vi "FlexMag - 23-03-2023.vi"() -> ()   [LabVIEW 2018] (continued)
                                n20029 = Greater?(x=w24311, y=0.0) -> (0:w24310:bool)
                                n20030 = case shown="True" w24310 {
                                frame False {
                                }
                                frame True {
                                n20031 = flat-sequence {
                                frame #0 {
                                n20032 = local read "R dc step length 5"() -> (w24318:dbl)
                                n20033 = local read "R dc step power 5"() -> (w24313:dbl)
                                n20034 = local read "R web speed"() -> (w24317:dbl)
                                n20035 = Divide(x=w24318, y=w24317) -> (x/y=w24316:dbl)
                                n20036 = Wait (ms)(milliseconds to wait=u32 100) -> ()  [unwired: 1 out]
                                n20037 = local write "Set DC Power ch2"(w24313) -> ()
                                n20038 = Multiply(x=w24316, y=60) -> (x*y=w24314:dbl)
                                n20039 = local write "time counting"(w24314) -> ()
                                }
                                frame #1 {
                                n20040 = local write "Dc_auto_set"(TRUE ("Dc_auto_set")) -> ()
                                }
                                frame #2 {
                                n20041 = while {
                                stop <- w24321 stop-if-true
                                n20042 = local read "time counting"() -> (w24327:dbl)
                                n20043 = local read "coating start"() -> (w24325:bool)
                                n20044 = Wait Until Next ms Multiple(millisecond multiple=u32 1000) -> ()  [unwired: 1 out]
                                n20045 = local read "abort ch2"() -> (w24323:bool)
                                n20046 = Decrement(x=w24327) -> (x-1=w24326:dbl)
                                n20047 = local write "time counting"(w24326) -> ()
                                n20048 = Not(x=w24325) -> (.not. x?=w24324:bool)
                                n20049 = Less Or Equal To 0?(x=w24326) -> (x <= 0?=w24322:bool)
                                n20050 = Compound Arithmetic op=OR(w24322, w24324, w24323) -> (w24321:bool)
                                }
                                }
                                }
                                }
                                }
                                }
                                }
                                }
                                frame True {
                                }
                                }
                                }
                                frame #5 {
                                n20051 = local read "abort ch2"() -> (w24328:bool)
                                n20052 = case shown="False" w24328 {
                                frame False {
                                n20053 = local read "coating start"() -> (w24329:bool)
                                n20054 = case shown="True" w24329 {
                                frame False {
                                }
                                frame True {
                                n20055 = local read "R dc step length 6"() -> (w24332:dbl)
                                n20056 = Greater?(x=w24332, y=0.0) -> (0:w24331:bool)
                                n20057 = case shown="True" w24331 {
                                frame False {
                                }
                                frame True {
                                n20058 = flat-sequence {
                                frame #0 {
                                n20059 = local read "R dc step length 6"() -> (w24339:dbl)
                                n20060 = local read "R dc step power 6"() -> (w24334:dbl)
                                n20061 = local read "R web speed"() -> (w24338:dbl)
                                n20062 = Wait (ms)(milliseconds to wait=u32 100) -> ()  [unwired: 1 out]
                                n20063 = Divide(x=w24339, y=w24338) -> (x/y=w24337:dbl)
                                n20064 = local write "Set DC Power ch2"(w24334) -> ()
                                n20065 = Multiply(x=w24337, y=60) -> (x*y=w24335:dbl)
                                n20066 = local write "time counting"(w24335) -> ()
                                }
                                frame #1 {
                                n20067 = local write "Dc_auto_set"(TRUE ("Dc_auto_set")) -> ()
                                }
                                frame #2 {
                                n20068 = while {
                                stop <- w24342 stop-if-true
                                n20069 = local read "time counting"() -> (w24348:dbl)
                                n20070 = local read "coating start"() -> (w24346:bool)
                                n20071 = local read "abort ch2"() -> (w24344:bool)
                                n20072 = Wait Until Next ms Multiple(millisecond multiple=u32 1000) -> ()  [unwired: 1 out]
                                n20073 = Decrement(x=w24348) -> (x-1=w24347:dbl)
                                n20074 = local write "time counting"(w24347) -> ()
                                n20075 = Not(x=w24346) -> (.not. x?=w24345:bool)
                                n20076 = Less Or Equal To 0?(x=w24347) -> (x <= 0?=w24343:bool)
                                n20077 = Compound Arithmetic op=OR(w24343, w24345, w24344) -> (w24342:bool)
                                }
                                }
                                }
                                }
                                }
                                }
                                }
                                }
                                frame True {
                                }
                                }
                                }
                                frame #6 {
                                n20078 = local read "abort ch2"() -> (w24349:bool)
                                n20079 = case shown="False" w24349 {
                                frame False {
                                n20080 = local read "coating start"() -> (w24350:bool)
                                n20081 = case shown="True" w24350 {
                                frame False {
                                }
                                frame True {
                                n20082 = local read "R dc step length 7"() -> (w24353:dbl)
                                n20083 = Greater?(x=w24353, y=0.0) -> (0:w24352:bool)
                                n20084 = case shown="True" w24352 {
                                frame False {
                                }
                                frame True {
                                n20085 = flat-sequence {
                                frame #0 {
                                n20086 = local read "R dc step length 7"() -> (w24360:dbl)
                                n20087 = local read "R dc step power 7"() -> (w24355:dbl)
                                n20088 = local read "R web speed"() -> (w24359:dbl)
                                n20089 = Divide(x=w24360, y=w24359) -> (x/y=w24358:dbl)
                                n20090 = Wait (ms)(milliseconds to wait=u32 100) -> ()  [unwired: 1 out]
                                n20091 = local write "Set DC Power ch2"(w24355) -> ()
                                n20092 = Multiply(x=w24358, y=60) -> (x*y=w24356:dbl)
                                n20093 = local write "time counting"(w24356) -> ()
                                }
                                frame #1 {
                                n20094 = local write "Dc_auto_set"(TRUE ("Dc_auto_set")) -> ()
                                }
                                frame #2 {
                                n20095 = while {
                                stop <- w24363 stop-if-true
                                n20096 = local read "time counting"() -> (w24369:dbl)
                                n20097 = local read "coating start"() -> (w24367:bool)
                                n20098 = local read "abort ch2"() -> (w24365:bool)
                                n20099 = Wait Until Next ms Multiple(millisecond multiple=u32 1000) -> ()  [unwired: 1 out]
                                n20100 = Decrement(x=w24369) -> (x-1=w24368:dbl)
                                n20101 = local write "time counting"(w24368) -> ()
                                n20102 = Not(x=w24367) -> (.not. x?=w24366:bool)
                                n20103 = Less Or Equal To 0?(x=w24368) -> (x <= 0?=w24364:bool)
                                n20104 = Compound Arithmetic op=OR(w24364, w24366, w24365) -> (w24363:bool)
                                }
                                }
                                }
                                }
                                }
                                }
                                }
                                }
                                frame True {
                                }
                                }
                                }
                                frame #7 {
                                n20105 = local read "abort ch2"() -> (w24370:bool)
                                n20106 = case shown="False" w24370 {
                                frame False {
                                n20107 = local read "coating start"() -> (w24371:bool)
                                n20108 = case shown="True" w24371 {
                                frame False {
                                }
                                frame True {
                                n20109 = local read "R dc step length 8"() -> (w24374:dbl)
                                n20110 = Greater?(x=w24374, y=0.0) -> (0:w24373:bool)
                                n20111 = case shown="True" w24373 {
                                frame False {
                                }
                                frame True {
                                n20112 = flat-sequence {
                                frame #0 {
                                n20113 = local read "R dc step length 8"() -> (w24381:dbl)
                                n20114 = local read "R dc step power 8"() -> (w24376:dbl)
                                n20115 = local read "R web speed"() -> (w24380:dbl)
                                n20116 = Wait (ms)(milliseconds to wait=u32 100) -> ()  [unwired: 1 out]
                                n20117 = Divide(x=w24381, y=w24380) -> (x/y=w24379:dbl)
                                n20118 = local write "Set DC Power ch2"(w24376) -> ()
                                n20119 = Multiply(x=w24379, y=60) -> (x*y=w24377:dbl)
                                n20120 = local write "time counting"(w24377) -> ()
                                }
                                frame #1 {
                                n20121 = local write "Dc_auto_set"(TRUE ("Dc_auto_set")) -> ()
                                }
                                frame #2 {
                                n20122 = while {
                                stop <- w24384 stop-if-true
                                n20123 = local read "time counting"() -> (w24390:dbl)
                                n20124 = local read "coating start"() -> (w24388:bool)
                                n20125 = Wait Until Next ms Multiple(millisecond multiple=u32 1000) -> ()  [unwired: 1 out]
                                n20126 = local read "abort ch2"() -> (w24386:bool)
                                n20127 = Decrement(x=w24390) -> (x-1=w24389:dbl)
                                n20128 = local write "time counting"(w24389) -> ()
                                n20129 = Not(x=w24388) -> (.not. x?=w24387:bool)
                                n20130 = Less Or Equal To 0?(x=w24389) -> (x <= 0?=w24385:bool)
                                n20131 = Compound Arithmetic op=OR(w24385, w24387, w24386) -> (w24384:bool)
                                }
                                }
                                }
                                }
                                }
                                }
                                }
                                }
                                frame True {
                                }
                                }
                                }
                                frame #8 {
                                n20132 = local read "abort ch2"() -> (w24391:bool)
                                n20133 = case shown="False" w24391 {
                                frame False {
                                n20134 = local read "coating start"() -> (w24392:bool)
                                n20135 = case shown="True" w24392 {
                                frame False {
                                }
                                frame True {
                                n20136 = local read "R dc step length 9"() -> (w24395:dbl)
                                n20137 = Greater?(x=w24395, y=0.0) -> (0:w24394:bool)
                                n20138 = case shown="True" w24394 {
                                frame False {
                                }
                                frame True {
                                n20139 = flat-sequence {
                                frame #0 {
                                n20140 = local read "R dc step length 9"() -> (w24402:dbl)
                                n20141 = local read "R dc step power 9"() -> (w24397:dbl)
                                n20142 = local read "R web speed"() -> (w24401:dbl)
                                n20143 = Wait (ms)(milliseconds to wait=u32 100) -> ()  [unwired: 1 out]
                                n20144 = Divide(x=w24402, y=w24401) -> (x/y=w24400:dbl)
                                n20145 = local write "Set DC Power ch2"(w24397) -> ()
                                n20146 = Multiply(x=w24400, y=60) -> (x*y=w24398:dbl)
                                n20147 = local write "time counting"(w24398) -> ()
                                }
                                frame #1 {
                                n20148 = local write "Dc_auto_set"(TRUE ("Dc_auto_set")) -> ()
                                }
                                frame #2 {
                                n20149 = while {
                                stop <- w24405 stop-if-true
                                n20150 = local read "time counting"() -> (w24411:dbl)
                                n20151 = local read "coating start"() -> (w24409:bool)
                                n20152 = local read "abort ch2"() -> (w24407:bool)
                                n20153 = Wait Until Next ms Multiple(millisecond multiple=u32 1000) -> ()  [unwired: 1 out]
                                n20154 = Decrement(x=w24411) -> (x-1=w24410:dbl)
                                n20155 = local write "time counting"(w24410) -> ()
                                n20156 = Not(x=w24409) -> (.not. x?=w24408:bool)
                                n20157 = Less Or Equal To 0?(x=w24410) -> (x <= 0?=w24406:bool)
                                n20158 = Compound Arithmetic op=OR(w24406, w24408, w24407) -> (w24405:bool)
                                }
                                }
                                }
                                }
                                }
                                }
                                }
                                }
                                frame True {
                                }
                                }
                                }
                                frame #9 {
                                n20159 = local read "abort ch2"() -> (w24412:bool)
                                n20160 = case shown="False" w24412 {
                                frame False {
                                n20161 = local read "coating start"() -> (w24413:bool)
                                n20162 = case shown="True" w24413 {
                                frame False {
                                }
                                frame True {
                                n20163 = local read "R dc step length 10"() -> (w24416:dbl)
                                n20164 = Greater?(x=w24416, y=0.0) -> (0:w24415:bool)
                                n20165 = case shown="True" w24415 {
                                frame False {
                                }
                                frame True {
                                n20166 = flat-sequence {
                                frame #0 {
                                n20167 = local read "R dc step length 10"() -> (w24423:dbl)
                                n20168 = local read "R dc step power 10"() -> (w24418:dbl)
                                n20169 = local read "R web speed"() -> (w24422:dbl)
                                n20170 = Divide(x=w24423, y=w24422) -> (x/y=w24421:dbl)
                                n20171 = local write "Set DC Power ch2"(w24418) -> ()
                                n20172 = Wait (ms)(milliseconds to wait=u32 100) -> ()  [unwired: 1 out]
                                n20173 = Multiply(x=w24421, y=60) -> (x*y=w24419:dbl)
                                n20174 = local write "time counting"(w24419) -> ()
                                }
                                frame #1 {
                                n20175 = local write "Dc_auto_set"(TRUE ("Dc_auto_set")) -> ()
                                }
                                frame #2 {
                                n20176 = while {
                                stop <- w24426 stop-if-true
                                n20177 = local read "time counting"() -> (w24432:dbl)
                                n20178 = local read "coating start"() -> (w24430:bool)
                                n20179 = local read "abort ch2"() -> (w24428:bool)
                                n20180 = Wait Until Next ms Multiple(millisecond multiple=u32 1000) -> ()  [unwired: 1 out]
                                n20181 = Decrement(x=w24432) -> (x-1=w24431:dbl)
                                n20182 = local write "time counting"(w24431) -> ()
                                n20183 = Not(x=w24430) -> (.not. x?=w24429:bool)
                                n20184 = Less Or Equal To 0?(x=w24431) -> (x <= 0?=w24427:bool)
                                n20185 = Compound Arithmetic op=OR(w24427, w24429, w24428) -> (w24426:bool)
                                }
                                }
                                }
                                }
                                }
                                }
                                }
                                }
                                frame True {
                                }
                                }
                                }
                                frame #10 {
                                n20186 = local read "abort ch2"() -> (w24433:bool)
                                n20187 = case shown="False" w24433 {
                                frame False {
                                n20188 = local read "coating start"() -> (w24434:bool)
                                n20189 = case shown="True" w24434 {
                                frame False {
                                }
                                frame True {
                                n20190 = Wait (ms)(milliseconds to wait=u32 100) -> ()  [unwired: 1 out]
                                "coating ch2 led 12" <- TRUE ("coating ch2 led 1")
                                }
                                }
                                }
                                frame True {
                                }
                                }
                                }
                                }
                                }
                                frame Enabled {
                                n20191 = stacked-sequence {
                                frame #0 {
                                n20192 = local read "abort ch2"() -> (w24437:bool)
                                n20193 = case shown="False" w24437 {
                                frame False {
                                n20194 = local read "coating start"() -> (w24438:bool)
                                n20195 = case shown="True" w24438 {
                                frame False {
                                }
                                frame True {
                                n20196 = local read "dep. for?"() -> (w24439:bool)
                                n20197 = case shown="True" w24439 {
                                frame False {
                                n20198 = flat-sequence {
                                frame #0 {
                                n20199 = local read "R DC number steps"() -> (w24442:dbl)
                                n20200 = case shown="10" w24442 {
                                tunnel: [0.0 ("step up") 1.0 ("step up") 2.0 ("step up") 3.0 ("step up") 4.0 ("step up") 5.0 ("step up") 6.0 ("step up") 7.0 ("step up") 8.0 ("step up") 9.0 ("step up") 10.0 ("step up") 11.0 ("step up") 12.0 ("step up") 13.0 ("step up") 14.0 ("step up") 15.0 ("step up") 16.0 ("step up") 17.0 ("step up") 18.0 ("step up") 19.0 ("step up") 20.0 ("step up")] -> w24441
                                tunnel: [200.0 ("R dc step power 1") w24447 w24449 w24451 w24453 w24455 w24457 w24459 w24461 w24463 w24465 w24467 w24469 w24471 w24473 w24475 w24477 w24479 w24481 w24483 w24485] -> w24440
                                frame 0, Default {
                                }
                                frame 1 {
                                n20201 = local read "R dc step power 1"() -> (w24447:dbl)
                                }
                                frame 2 {
                                n20202 = local read "R dc step power 2"() -> (w24449:dbl)
                                }
                                frame 3 {
                                n20203 = local read "R dc step power 3"() -> (w24451:dbl)
                                }
                                frame 4 {
                                n20204 = local read "R dc step power 4"() -> (w24453:dbl)
                                }
                                frame 5 {
                                n20205 = local read "R dc step power 5"() -> (w24455:dbl)
                                }
                                frame 6 {
                                n20206 = local read "R dc step power 6"() -> (w24457:dbl)
                                }
                                frame 7 {
                                n20207 = local read "R dc step power 7"() -> (w24459:dbl)
                                }
                                frame 8 {
                                n20208 = local read "R dc step power 8"() -> (w24461:dbl)
                                }
                                frame 9 {
                                n20209 = local read "R dc step power 9"() -> (w24463:dbl)
                                }
                                frame 10 {
                                n20210 = local read "R dc step power 10"() -> (w24465:dbl)
                                }
                                frame 11 {
                                n20211 = local read "R dc step power 11"() -> (w24467:dbl)
                                }
                                frame 12 {
                                n20212 = local read "R dc step power 12"() -> (w24469:dbl)
                                }
                                frame 13 {
                                n20213 = local read "R dc step power 13"() -> (w24471:dbl)
                                }
                                frame 14 {
                                n20214 = local read "R dc step power 14"() -> (w24473:dbl)
                                }
                                frame 15 {
                                n20215 = local read "R dc step power 15"() -> (w24475:dbl)
                                }
                                frame 16 {
                                n20216 = local read "R dc step power 16"() -> (w24477:dbl)
                                }
                                frame 17 {
                                n20217 = local read "R dc step power 17"() -> (w24479:dbl)
                                }
                                frame 18 {
                                n20218 = local read "R dc step power 18"() -> (w24481:dbl)
                                }
                                frame 19 {
                                n20219 = local read "R dc step power 19"() -> (w24483:dbl)
                                }
                                frame 20 {
                                n20220 = local read "R dc step power 20"() -> (w24485:dbl)
                                }
                                }
                                n20221 = Wait (ms)(milliseconds to wait=u32 100) -> ()  [unwired: 1 out]
                                n20222 = local write "current step"(w24441) -> ()
                                n20223 = local write "Set DC Power auto"(w24440) -> ()
                                }
                                frame #1 {
                                n20224 = local write "Dc_auto_set"(TRUE ("Dc_auto_set")) -> ()
                                }
                                frame #2 {
                                n20225 = Wait (ms)(milliseconds to wait=u32 1000) -> ()  [unwired: 1 out]
                                }
                                }
                                }
                                frame True {
                                n20226 = flat-sequence {
                                frame #0 {
                                n20227 = local read "R dc step power 1"() -> (w24490:dbl)
                                n20228 = Wait (ms)(milliseconds to wait=u32 100) -> ()  [unwired: 1 out]
                                n20229 = local write "Set DC Power auto"(w24490) -> ()
                                n20230 = local write "current step"(1.0 ("step up")) -> ()
                                }
                                frame #1 {
                                n20231 = local write "Dc_auto_set"(TRUE ("Dc_auto_set")) -> ()
                                }
                                frame #2 {
                                n20232 = Wait (ms)(milliseconds to wait=u32 1000) -> ()  [unwired: 1 out]
                                }
                                }
                                }
                                }
                                }
                                }
                                }
                                frame True {
                                }
                                }
                                }
                                frame #1 {
                                n20233 = local read "abort ch2"() -> (w24493:bool)
                                n20234 = case shown="False" w24493 {
                                frame False {
                                n20235 = local read "coating start"() -> (w24494:bool)
                                n20236 = case shown="True" w24494 {
                                frame False {
                                }
                                frame True {
                                n20237 = while {
                                i -> [w24495]
                                stop <- w24507 stop-if-true
                                n20238 = local read "step count"() -> (w24510:dbl)
                                n20239 = local read "R DC number steps"() -> (w24508:dbl)
                                n20240 = local read "roll error (min)"() -> (w24498:i32)
                                n20241 = Wait Until Next ms Multiple(millisecond multiple=u32 300) -> ()  [unwired: 1 out]
                                n20242 = feedback #340() -> (w24511:dbl)  [unwired: 1 in]
                                n20243 = feedback-in #340(w24510) -> ()
                                n20244 = Multiply(x=200, y=w24498) -> (x*y=w24499:i32)
                                n20245 = Less?(x=w24510, y=w24511) -> (x < y?=w24509:bool)
                                n20246 = case shown="True" w24509 {
                                tunnel: w24508 -> [_ w24518]
                                tunnel: [FALSE w24515] -> w24501
                                frame False {
                                }
                                frame True {
                                n20247 = local read "current step"() -> (w24517:dbl)
                                n20248 = Greater Or Equal?(x=w24518, y=w24517) -> (x >= y?=w24516:bool)
                                n20249 = Not(x=w24516) -> (.not. x?=w24515:bool)
                                n20250 = case shown="True" w24516 {
                                tunnel: w24517 -> [_ w24519]
                                frame False {
                                }
                                frame True {
                                n20251 = case shown="4" w24519 {
                                frame 0, Default {
                                }
                                frame 1 {
                                n20252 = stacked-sequence {
                                frame #0 {
                                n20253 = local read "R dc step power 1"() -> (w24521:dbl)
                                n20254 = local write "Set DC Power auto"(w24521) -> ()
                                n20255 = Wait (ms)(milliseconds to wait=u32 100) -> ()  [unwired: 1 out]
                                }
                                frame #1 {
                                n20256 = local write "Dc_auto_set"(TRUE ("Dc_auto_set")) -> ()
                                }
                                }
                                }
                                frame 2 {
                                n20257 = stacked-sequence {
                                frame #0 {
                                n20258 = local read "R dc step power 2"() -> (w24524:dbl)
                                n20259 = local write "Set DC Power auto"(w24524) -> ()
                                n20260 = Wait (ms)(milliseconds to wait=u32 100) -> ()  [unwired: 1 out]
                                }
                                frame #1 {
                                n20261 = local write "Dc_auto_set"(TRUE ("Dc_auto_set")) -> ()
                                }
                                }
                                }
                                frame 3 {
                                n20262 = stacked-sequence {
                                frame #0 {
                                n20263 = local read "R dc step power 3"() -> (w24527:dbl)
                                n20264 = local write "Set DC Power auto"(w24527) -> ()
                                n20265 = Wait (ms)(milliseconds to wait=u32 100) -> ()  [unwired: 1 out]
                                }
                                frame #1 {
                                n20266 = local write "Dc_auto_set"(TRUE ("Dc_auto_set")) -> ()
                                }
                                }
                                }
                                frame 4 {
                                n20267 = stacked-sequence {
                                frame #0 {
                                n20268 = local read "R dc step power 4"() -> (w24530:dbl)
                                n20269 = local write "Set DC Power auto"(w24530) -> ()
                                n20270 = Wait (ms)(milliseconds to wait=u32 100) -> ()  [unwired: 1 out]
                                }
                                frame #1 {
                                n20271 = local write "Dc_auto_set"(TRUE ("Dc_auto_set")) -> ()
                                }
                                }
                                }
                                frame 5 {
                                n20272 = stacked-sequence {
                                frame #0 {
                                n20273 = local read "R dc step power 5"() -> (w24533:dbl)
                                n20274 = local write "Set DC Power auto"(w24533) -> ()
                                n20275 = Wait (ms)(milliseconds to wait=u32 100) -> ()  [unwired: 1 out]
                                }
                                frame #1 {
                                n20276 = local write "Dc_auto_set"(TRUE ("Dc_auto_set")) -> ()
                                }
                                }
                                }
                                frame 6 {
                                n20277 = stacked-sequence {
                                frame #0 {
                                n20278 = local read "R dc step power 6"() -> (w24536:dbl)
                                n20279 = local write "Set DC Power auto"(w24536) -> ()
                                n20280 = Wait (ms)(milliseconds to wait=u32 100) -> ()  [unwired: 1 out]
                                }
                                frame #1 {
                                n20281 = local write "Dc_auto_set"(TRUE ("Dc_auto_set")) -> ()
                                }
                                }
                                }
                                frame 7 {
                                n20282 = stacked-sequence {
                                frame #0 {
                                n20283 = local read "R dc step power 7"() -> (w24539:dbl)
                                n20284 = local write "Set DC Power auto"(w24539) -> ()
                                n20285 = Wait (ms)(milliseconds to wait=u32 100) -> ()  [unwired: 1 out]
                                }
                                frame #1 {
                                n20286 = local write "Dc_auto_set"(TRUE ("Dc_auto_set")) -> ()
                                }
                                }
                                }
                                frame 8 {
                                n20287 = stacked-sequence {
                                frame #0 {
                                n20288 = local read "R dc step power 8"() -> (w24542:dbl)
                                n20289 = local write "Set DC Power auto"(w24542) -> ()
                                n20290 = Wait (ms)(milliseconds to wait=u32 100) -> ()  [unwired: 1 out]
                                }
                                frame #1 {
                                n20291 = local write "Dc_auto_set"(TRUE ("Dc_auto_set")) -> ()
                                }
                                }
                                }
                                frame 9 {
                                n20292 = stacked-sequence {
                                frame #0 {
                                n20293 = local read "R dc step power 9"() -> (w24545:dbl)
                                n20294 = local write "Set DC Power auto"(w24545) -> ()
                                n20295 = Wait (ms)(milliseconds to wait=u32 100) -> ()  [unwired: 1 out]
                                }
                                frame #1 {
                                n20296 = local write "Dc_auto_set"(TRUE ("Dc_auto_set")) -> ()
                                }
                                }
                                }
                                frame 10 {
                                n20297 = stacked-sequence {
                                frame #0 {
                                n20298 = local read "R dc step power 10"() -> (w24548:dbl)
                                n20299 = local write "Set DC Power auto"(w24548) -> ()
                                n20300 = Wait (ms)(milliseconds to wait=u32 100) -> ()  [unwired: 1 out]
                                }
                                frame #1 {
                                n20301 = local write "Dc_auto_set"(TRUE ("Dc_auto_set")) -> ()
                                }
                                }
                                }
                                frame 11 {
                                n20302 = stacked-sequence {
                                frame #0 {
                                n20303 = local read "R dc step power 11"() -> (w24551:dbl)
                                n20304 = local write "Set DC Power auto"(w24551) -> ()
                                n20305 = Wait (ms)(milliseconds to wait=u32 100) -> ()  [unwired: 1 out]
                                }
                                frame #1 {
                                n20306 = local write "Dc_auto_set"(TRUE ("Dc_auto_set")) -> ()
                                }
                                }
                                }
                                frame 12 {
                                n20307 = stacked-sequence {
                                frame #0 {
                                n20308 = local read "R dc step power 12"() -> (w24554:dbl)
                                n20309 = local write "Set DC Power auto"(w24554) -> ()
                                n20310 = Wait (ms)(milliseconds to wait=u32 100) -> ()  [unwired: 1 out]
                                }
                                frame #1 {
                                n20311 = local write "Dc_auto_set"(TRUE ("Dc_auto_set")) -> ()
                                }
                                }
                                }
                                frame 13 {
                                n20312 = stacked-sequence {
                                frame #0 {
                                n20313 = local read "R dc step power 13"() -> (w24557:dbl)
                                n20314 = local write "Set DC Power auto"(w24557) -> ()
                                n20315 = Wait (ms)(milliseconds to wait=u32 100) -> ()  [unwired: 1 out]
                                }
                                frame #1 {
                                n20316 = local write "Dc_auto_set"(TRUE ("Dc_auto_set")) -> ()
                                }
                                }
                                }
                                frame 14 {
                                n20317 = stacked-sequence {
                                frame #0 {
                                n20318 = local read "R dc step power 14"() -> (w24560:dbl)
                                n20319 = local write "Set DC Power auto"(w24560) -> ()
                                n20320 = Wait (ms)(milliseconds to wait=u32 100) -> ()  [unwired: 1 out]
                                }
                                frame #1 {
                                n20321 = local write "Dc_auto_set"(TRUE ("Dc_auto_set")) -> ()
                                }
                                }
                                }
                                frame 15 {
                                n20322 = stacked-sequence {
                                frame #0 {
                                n20323 = local read "R dc step power 15"() -> (w24563:dbl)
                                n20324 = local write "Set DC Power auto"(w24563) -> ()
                                n20325 = Wait (ms)(milliseconds to wait=u32 100) -> ()  [unwired: 1 out]
                                }
                                frame #1 {
                                n20326 = local write "Dc_auto_set"(TRUE ("Dc_auto_set")) -> ()
                                }
                                }
                                }
                                frame 16 {
                                n20327 = stacked-sequence {
                                frame #0 {
                                n20328 = local read "R dc step power 16"() -> (w24566:dbl)
                                n20329 = local write "Set DC Power auto"(w24566) -> ()
                                n20330 = Wait (ms)(milliseconds to wait=u32 100) -> ()  [unwired: 1 out]
                                }
                                frame #1 {
                                n20331 = local write "Dc_auto_set"(TRUE ("Dc_auto_set")) -> ()
                                }
                                }
                                }
                                frame 17 {
                                n20332 = stacked-sequence {
                                frame #0 {
                                n20333 = local read "R dc step power 17"() -> (w24569:dbl)
                                n20334 = local write "Set DC Power auto"(w24569) -> ()
                                n20335 = Wait (ms)(milliseconds to wait=u32 100) -> ()  [unwired: 1 out]
                                }
                                frame #1 {
                                n20336 = local write "Dc_auto_set"(TRUE ("Dc_auto_set")) -> ()
                                }
                                }
                                }
                                frame 18 {
                                n20337 = stacked-sequence {
                                frame #0 {
                                n20338 = local read "R dc step power 18"() -> (w24572:dbl)
                                n20339 = local write "Set DC Power auto"(w24572) -> ()
                                n20340 = Wait (ms)(milliseconds to wait=u32 100) -> ()  [unwired: 1 out]
                                }
                                frame #1 {
                                n20341 = local write "Dc_auto_set"(TRUE ("Dc_auto_set")) -> ()
                                }
                                }
                                }
                                frame 19 {
                                n20342 = stacked-sequence {
                                frame #0 {
                                n20343 = local read "R dc step power 19"() -> (w24575:dbl)
                                n20344 = local write "Set DC Power auto"(w24575) -> ()
                                n20345 = Wait (ms)(milliseconds to wait=u32 100) -> ()  [unwired: 1 out]
                                }
                                frame #1 {
                                n20346 = local write "Dc_auto_set"(TRUE ("Dc_auto_set")) -> ()
                                }
                                }
                                }
                                frame 20 {
                                n20347 = stacked-sequence {
                                frame #0 {
                                n20348 = local read "R dc step power 20"() -> (w24578:dbl)
                                n20349 = local write "Set DC Power auto"(w24578) -> ()
                                n20350 = Wait (ms)(milliseconds to wait=u32 100) -> ()  [unwired: 1 out]
                                }
                                frame #1 {
                                n20351 = local write "Dc_auto_set"(TRUE ("Dc_auto_set")) -> ()
                                }
                                }
                                }
                                }
                                }
                                }
                                }
                                }
                                n20352 = Greater?(x=w24495, y=w24499) -> (0:w24497:bool)
                                n20353 = case shown="True" w24497 {
                                frame False {
                                }
                                frame True {
                                n20354 = local write "Warning Message"("Automatic Coating Process is canceled !\nCH2  rolling problem..." ("Warning Message")) -> ()
                                n20355 = local write "coating error"(TRUE ("coating error")) -> ()
                                }
                                }
                                n20356 = local read "CH2_Motor DO"() -> (w24503:bool)
                                n20357 = local read "coating start"() -> (w24506:bool)
                                n20358 = local read "abort ch2"() -> (w24504:bool)
                                n20359 = Not(x=w24503) -> (.not. x?=w24502:bool)
                                n20360 = Not(x=w24506) -> (.not. x?=w24505:bool)
                                n20361 = Compound Arithmetic op=OR(w24501, w24502, w24504, w24505) -> (w24507:bool)
                                }
                                }
                                }
                                }
                                frame True {
                                }
                                }
                                }
                                }
                                }
                                }
                                }
                                frame #13 {
                                # "DC off"
                                n20362 = stacked-sequence {
                                frame #0 {
                                n20363 = local read "abort ch2"() -> (w24580:bool)
                                n20364 = case shown="False" w24580 {
                                frame False {
                                n20365 = local read "coating start"() -> (w24581:bool)
                                n20366 = case shown="True" w24581 {
                                frame False {
                                }
                                frame True {
                                n20367 = stacked-sequence {
                                frame #0 {
                                n20368 = Wait (ms)(milliseconds to wait=u32 1000) -> ()  [unwired: 1 out]
                                }
                                frame #1 {
                                n20369 = flat-sequence {
                                frame #0 {
                                n20370 = local write "Dc_auto_off"(TRUE ("Dc_auto_off")) -> ()
                                }
                                frame #1 {
                                n20371 = local write "Set DC Power auto"(0.0 ("Set DC Power")) -> ()
                                n20372 = local write "Dc_auto_off"(FALSE ("Dc_auto_off")) -> ()
                                n20373 = Wait (ms)(milliseconds to wait=u32 2000) -> ()  [unwired: 1 out]
                                }
                                frame #2 {
                                n20374 = local write "Dc_auto_off"(TRUE ("Dc_auto_off")) -> ()
                                }
                                frame #3 {
                                n20375 = Wait (ms)(milliseconds to wait=u32 1000) -> ()  [unwired: 1 out]
                                }
                                }
                                }
                                }
                                }
                                }
                                }
                                frame True {
                                }
                                }
                                }
                                frame #1 {
                                n20376 = local read "abort ch2"() -> (w24589:bool)
                                n20377 = case shown="False" w24589 {
                                frame False {
                                n20378 = local read "coating start"() -> (w24590:bool)
                                n20379 = case shown="True" w24590 {
                                frame False {
                                }
                                frame True {
                                n20380 = while {
                                i -> [w24593]
                                stop <- w24595 stop-if-true
                                n20381 = Greater Or Equal?(x=w24593, y=10) -> (x >= y?=w24594:bool)
                                n20382 = case shown="True" w24594 {
                                frame False {
                                }
                                frame True {
                                n20383 = local write "Warning Message"("Automatic Coating Process is canceled !\nDCPS cannot be turned off." ("Warning Message")) -> ()
                                n20384 = local write "coating error"(TRUE ("coating error")) -> ()
                                }
                                }
                                n20385 = local read "Dcps_is_on"() -> (w24599:bool)
                                n20386 = case shown="True" w24599 {
                                tunnel: [TRUE ("CH2_WFC_DO") FALSE ("CH2_WFC_DO")] -> w24598
                                frame False {
                                }
                                frame True {
                                n20387 = Wait Until Next ms Multiple(millisecond multiple=u32 1000) -> ()  [unwired: 1 out]
                                n20388 = local write "Dc_auto_off"(TRUE ("coating error")) -> ()
                                }
                                }
                                n20389 = local read "coating start"() -> (w24597:bool)
                                n20390 = local read "abort ch2"() -> (w24591:bool)
                                n20391 = Not(x=w24597) -> (.not. x?=w24596:bool)
                                n20392 = Compound Arithmetic op=OR(w24598, w24596, w24591) -> (w24595:bool)
                                }
                                }
                                }
                                }
                                frame True {
                                }
                                }
                                }
                                frame #2 {
                                n20393 = local read "abort ch2"() -> (w24606:bool)
                                n20394 = case shown="False" w24606 {
                                frame False {
                                n20395 = local read "coating start"() -> (w24607:bool)
                                n20396 = case shown="True" w24607 {
                                frame False {
                                }
                                frame True {
                                n20397 = Wait (ms)(milliseconds to wait=u32 100) -> ()  [unwired: 1 out]
                                "coating ch2 led 13" <- TRUE ("coating ch2 led 1")
                                }
                                }
                                }
                                frame True {
                                }
                                }
                                }
                                }
                                }
                                frame #14 {
                                # "pcgv open"
                                n20398 = stacked-sequence {
                                frame #0 {
                                n20399 = local read "abort ch2"() -> (w24610:bool)
                                n20400 = case shown="False" w24610 {
                                frame False {
                                n20401 = local read "coating start"() -> (w24611:bool)
                                n20402 = case shown="True" w24611 {
                                frame False {
                                }
                                frame True {
                                n20403 = local write "pcgv2 auto open"(TRUE ("ch3 ar set zero auto")) -> ()
                                }
                                }
                                }
                                frame True {
                                }
                                }
                                }
                                frame #1 {
                                n20404 = local read "abort ch2"() -> (w24613:bool)
                                n20405 = case shown="False" w24613 {
                                frame False {
                                n20406 = local read "coating start"() -> (w24614:bool)
                                n20407 = case shown="True" w24614 {
                                frame False {
                                }
                                frame True {
                                n20408 = while {
                                i -> [w24618]
                                stop <- w24620 stop-if-true
                                n20409 = Greater Or Equal?(x=w24618, y=50) -> (x >= y?=w24619:bool)
                                n20410 = case shown="True" w24619 {
                                frame False {
                                }
                                frame True {
                                n20411 = local write "Warning Message"("Automatic Coating Process is canceled !\nCH2 PCGV couldn't be opened..." ("Warning Message")) -> ()
                                n20412 = local write "coating error"(TRUE ("coating error")) -> ()
                                }
                                }
                                n20413 = local read "ch2_pcgv_gui"() -> (w24615:bool)
                                n20414 = case shown="False" w24615 {
                                tunnel: [FALSE ("CH2_WFC_DO") TRUE ("CH2_WFC_DO")] -> w24623
                                frame False {
                                n20415 = Wait Until Next ms Multiple(millisecond multiple=u32 1000) -> ()  [unwired: 1 out]
                                n20416 = local write "pcgv2 auto open"(TRUE ("coating error")) -> ()
                                }
                                frame True {
                                }
                                }
                                n20417 = local read "coating start"() -> (w24622:bool)
                                n20418 = local read "abort ch2"() -> (w24616:bool)
                                n20419 = Not(x=w24622) -> (.not. x?=w24621:bool)
                                n20420 = Compound Arithmetic op=OR(w24623, w24621, w24616) -> (w24620:bool)
                                }
                                }
                                }
                                }
                                frame True {
                                }
                                }
                                }
                                frame #2 {
                                n20421 = local read "abort ch2"() -> (w24630:bool)
                                n20422 = case shown="False" w24630 {
                                frame False {
                                n20423 = local read "coating start"() -> (w24631:bool)
                                n20424 = case shown="True" w24631 {
                                frame False {
                                }
                                frame True {
                                n20425 = Wait (ms)(milliseconds to wait=u32 100) -> ()  [unwired: 1 out]
                                "coating ch2 led 14" <- TRUE ("coating ch2 led 1")
                                }
                                }
                                }
                                frame True {
                                }
                                }
                                }
                                }
                                }
                                frame #15 {
                                # "argon set zero"
                                n20426 = stacked-sequence {
                                frame #0 {
                                n20427 = local read "abort ch2"() -> (w24634:bool)
                                n20428 = case shown="False" w24634 {
                                frame False {
                                n20429 = local read "coating start"() -> (w24635:bool)
                                n20430 = case shown="True" w24635 {
                                frame False {
                                }
                                frame True {
                                n20431 = local write "ch2 ar set zero auto"(TRUE ("ch3 ar set zero auto")) -> ()
                                }
                                }
                                }
                                frame True {
                                }
                                }